vi "UHR-Fleezers Control (host) - 12.6.1.vi"() -> ()   [LabVIEW 2012] (continued)
                    n401 = property on="Saved AOD Raster Scan Parameter Sets" class="Arr (strict)"("Index Values"=w674) -> ()  [unwired: 2 in, 2 out]
                  }
                  frame #1 {
                    n402 = Wait (ms)(milliseconds to wait=u32 200) -> ()  [unwired: 1 out]
                  }
                  frame #2 {
                    n403 = property on="Load parameters" class="Bool (strict)"("Val(Sgnl)"=TRUE ("Value (Signaling)")) -> ()  [unwired: 2 in, 2 out]
                  }
                  frame #3 {
                    n404 = Wait (ms)(milliseconds to wait=u32 200) -> ()  [unwired: 1 out]
                  }
                  frame #4 {
                    n405 = property on="Trap Raster Scan" class="Bool (strict)"("Val(Sgnl)"=TRUE ("Value (Signaling)")) -> ()  [unwired: 2 in, 2 out]
                  }
                  frame #5 {
                    n406 = Wait (ms)(milliseconds to wait=u32 2000) -> ()  [unwired: 1 out]
                  }
                  frame #6 {
                    n407 = while {
                      stop <- w687 stop-if-true
                      n408 = local read "Raster Scanning..."() -> (w689:bool)
                      n409 = local read "Saving..."() -> (w685:bool)
                      n410 = Wait (ms)(milliseconds to wait=u32 100) -> ()  [unwired: 1 out]
                      n411 = Not(x=w685) -> (.not. x?=w684:bool)
                      n412 = Not(x=w689) -> (.not. x?=w686:bool)
                      n413 = And(x=w686, y=w684) -> (x .and. y?=w687:bool)
                    }
                  }
                  frame #7 {
                    n414 = property on="Trap Delta (MHz)" class="DigNum (strict)"("Val(Sgnl)"=w690) -> ()  [unwired: 2 in, 2 out]
                  }
                }
              }
            }
          }
          frame #8 {
            n415 = local read "Save ave N"() -> (w692:dbl)
            n416 = case shown="False" "W/ Offset 2" {
              tunnel: w693 -> [_ w700]
              tunnel: w692 -> [_ w699]
              tunnel: w691 -> [w695 _]
              frame False {
                n417 = case shown="False" w695 {
                  frame False {
                    n418 = Multiply(x="Cal read wait (s)", y=u32 1000 ("milliseconds to wait")) -> (x*y=w697:u32)
                    n419 = Wait (ms)(milliseconds to wait=w697) -> ()  [unwired: 1 out]
                  }
                  frame True {
                  }
                }
              }
              frame True {
                n420 = stacked-sequence {
                  tunnel: w700 -> [_ _ _ _ _ _ _ _ _ w721 _ _]
                  tunnel: w699 -> [_ _ _ _ _ _ _ _ _ w719 _ _]
                  frame #0 {
                    n421 = property on="Save ave N" class="DigNum (strict)"("Val(Sgnl)"=1.0 ("Value (Signaling)")) -> ()  [unwired: 2 in, 2 out]
                  }
                  frame #1 {
                    n422 = Wait (ms)(milliseconds to wait=u32 500) -> ()  [unwired: 1 out]
                  }
                  frame #2 {
                    n423 = property on="Trap Delta (MHz)" class="DigNum (strict)"("Val(Sgnl)"="Offset 2 Start (MHz)") -> ()  [unwired: 2 in, 2 out]
                    n424 = Replace Array Subset(array=u32[] [0] ("Index Values"), new element="Offset 2 Set", index=0) -> (w705:u32[])
                    n425 = property on="Saved AOD Raster Scan Parameter Sets" class="Arr (strict)"("Index Values"=w705) -> ()  [unwired: 2 in, 2 out]
                  }
                  frame #3 {
                    n426 = Wait (ms)(milliseconds to wait=u32 500) -> ()  [unwired: 1 out]
                  }
                  frame #4 {
                    n427 = property on="Load parameters" class="Bool (strict)"("Val(Sgnl)"=TRUE ("Value (Signaling)")) -> ()  [unwired: 2 in, 2 out]
                  }
                  frame #5 {
                    n428 = Wait (ms)(milliseconds to wait=u32 500) -> ()  [unwired: 1 out]
                  }
                  frame #6 {
                    n429 = property on="Trap Raster Scan" class="Bool (strict)"("Val(Sgnl)"=TRUE ("Value (Signaling)")) -> ()  [unwired: 2 in, 2 out]
                  }
                  frame #7 {
                    n430 = Wait (ms)(milliseconds to wait=u32 2000) -> ()  [unwired: 1 out]
                  }
                  frame #8 {
                    n431 = while {
                      stop <- w714 stop-if-true
                      n432 = local read "Raster Scanning..."() -> (w717:bool)
                      n433 = local read "Saving..."() -> (w715:bool)
                      n434 = Wait (ms)(milliseconds to wait=u32 100) -> ()  [unwired: 1 out]
                      n435 = Not(x=w715) -> (.not. x?=w713:bool)
                      n436 = Not(x=w717) -> (.not. x?=w716:bool)
                      n437 = And(x=w716, y=w713) -> (x .and. y?=w714:bool)
                    }
                  }
                  frame #9 {
                    n438 = property on="Trap Delta (MHz)" class="DigNum (strict)"("Val(Sgnl)"=w721) -> ()  [unwired: 2 in, 2 out]
                    n439 = property on="Saved AOD Raster Scan Parameter Sets" class="Arr (strict)"("Index Values"=u32[] [0]) -> ()  [unwired: 2 in, 2 out]
                    n440 = property on="Save ave N" class="DigNum (strict)"("Val(Sgnl)"=w719) -> ()  [unwired: 2 in, 2 out]
                  }
                  frame #10 {
                    n441 = Wait (ms)(milliseconds to wait=u32 500) -> ()  [unwired: 1 out]
                  }
                  frame #11 {
                    n442 = property on="Load parameters" class="Bool (strict)"("Val(Sgnl)"=TRUE ("Value (Signaling)")) -> ()  [unwired: 2 in, 2 out]
                  }
                }
              }
            }
          }
          frame #9 {
            n443 = property on="Read Cal" class="Bool (strict)"("Val(Sgnl)"=TRUE ("Value (Signaling)")) -> ()  [unwired: 2 in, 2 out]
          }
          frame #10 {
            n444 = Wait (ms)(milliseconds to wait=u32 1000) -> ()  [unwired: 1 out]
          }
          frame #11 {
            n445 = property on="Fish for Tether" class="Bool (strict)"("Val(Sgnl)"=TRUE ("Value (Signaling)")) -> ()  [unwired: 2 in, 2 out]
          }
        }
        n446 = local write "Cal/Data Acq. Spot"(FALSE ("Cal/Data Acq. Spot")) -> ()
      }
      event "Dump Beads": Value Change {
        n447 = event-data() -> ()  [unwired: 1 in, 5 out]
        n448 = flat-sequence {
          tunnel: ["Dump spot flow on?"] -> w727
          tunnel: [w738] -> w728
          tunnel: w727 -> [w738]
          tunnel: w731 -> [w743]
          tunnel: w730 -> [w742]
          tunnel: [w740] -> w729
          tunnel: w728 -> [w740]
          tunnel: w729 -> [w753]
          frame #0 {
            w732 = FALSE ("Value (Signaling)")
            n449 = local read "Saving..."() -> (w734:bool)
            n450 = local write "Dump Beads"(FALSE ("Dump Beads")) -> ()
            n451 = property on="Inject Pump 3" class="Bool (strict)"("Val(Sgnl)"=w732) -> ()  [unwired: 2 in, 2 out]
            n452 = property on="Inject Pump 1" class="Bool (strict)"("Val(Sgnl)"=w732) -> ()  [unwired: 2 in, 2 out]
            n453 = local write "Stop Saving"(w734) -> ()
          }
          frame #1 {
            w735 = FALSE ("Fl. Triggered...")
            n454 = case shown="True" "Dump spot flow on?" {
              frame False {
              }
              frame True {
                n455 = property on="Sample Channel\nFlow" class="Bool (strict)"("Val(Sgnl)"=TRUE ("Stage Moving")) -> ()  [unwired: 2 in, 2 out]
              }
            }
            n456 = local write "Fl. Triggered..."(w735) -> ()
            n457 = local write "Tether"(w735) -> ()
            n458 = property on="Green Laser ON" class="Bool (strict)"("Val(Sgnl)"=w735) -> ()  [unwired: 2 in, 2 out]
            n459 = property on="Trap Pos. FB ON" class="Bool (strict)"("Val(Sgnl)"=w735) -> ()  [unwired: 2 in, 2 out]
            n460 = property on="Trap Trig. Fl." class="Bool (strict)"("Val(Sgnl)"=w735) -> ()  [unwired: 2 in, 2 out]
            n461 = property on="Fl. Triggered..." class="Bool (strict)"("Val(Sgnl)"=w735) -> ()  [unwired: 2 in, 2 out]
            n462 = property on="Dip for Protein" class="Bool (strict)"("Val(Sgnl)"=w735) -> ()  [unwired: 2 in, 2 out]
            n463 = property on="Pause dwell" class="Bool (strict)"("Val(Sgnl)"=w735) -> ()  [unwired: 2 in, 2 out]
          }
          frame #2 {
            n464 = property on="Trap Pos. FB Offset Factor" class="DigNum (strict)"("Val(Sgnl)"=i64 0 ("Value (Signaling)")) -> ()  [unwired: 2 in, 2 out]
          }
          frame #3 {
            n465 = local read "Saved Stage Positions"() -> (w744:dbl[][])
            n466 = local write "Stage Moving"(TRUE ("Stage Moving")) -> ()
            n467 = Array Subset(array=w744, index (row)=3 ("index"), length (row)=1 ("length"), index (col)=1 ("index"), length (col)=3 ("length")) -> (w749:dbl[][])
            n468 = Reshape Array(w749, 3 ("dimension size")) -> (w747:dbl[])
            n469 = Array To Cluster(array=w747) -> (cluster=w746:cluster{"[0]":dbl, "[1]":dbl, "[2]":dbl})
            n470 = call "Set Stage Position.vi"("Position"=w746, "error in"=w742, "VISA resource name in"=w743) -> ()  [unwired: 3 out]
          }
          frame #4 {
            w754 = FALSE ("Value (Signaling)")
            n471 = case shown="True" w753 {
              frame False {
              }
              frame True {
                n472 = property on="Sample Channel\nFlow" class="Bool (strict)"("Val(Sgnl)"=FALSE ("Stage Moving")) -> ()  [unwired: 2 in, 2 out]
              }
            }
            n473 = property on="Trap 1 (ON/OFF)" class="Bool (strict)"("Val(Sgnl)"=w754) -> ()  [unwired: 2 in, 2 out]
            n474 = property on="Trap 2 (ON/OFF)" class="Bool (strict)"("Val(Sgnl)"=w754) -> ()  [unwired: 2 in, 2 out]
            n475 = call <vilib>:"Beep.vi"() -> ()  [unwired: 3 in, 9 out]
          }
          frame #5 {
            n476 = property on="Move Cap. 2 (ADig Top)" class="Bool (strict)"("Val(Sgnl)"=TRUE ("Value (Signaling)")) -> ()  [unwired: 2 in, 2 out]
            n477 = property on="Tab Control" class="TabCtl (strict)"("Val(Sgnl)"=T26."Status" ("Value (Signaling)")) -> ()  [unwired: 2 in, 2 out]
          }
        }
      }
      event "Dip for Protein": Value Change {
        n478 = event-data() -> ()  [unwired: 1 in, 5 out]
        n479 = case shown="True" "Dip for Protein" {
          tunnel: w760 -> [_ w762]
          tunnel: w759 -> [_ w761]
          frame False {
          }
          frame True {
            n480 = while {
              tunnel: w762 -> [w773]
              tunnel: w761 -> [w772]
              i -> [w767]
              stop <- w769 stop-if-true
              n481 = Increment(x=w767) -> (x+1=→"Dip #":i32)
              n482 = flat-sequence {
                tunnel: w772 -> [w784]
                tunnel: w773 -> [w785]
                tunnel: [w785] -> w777
                tunnel: [w784] -> w776
                tunnel: [w778] -> w763
                tunnel: [w790] -> w771
                tunnel: [w791] -> w770
                tunnel: w777 -> [w792]
                tunnel: w776 -> [w793]
                tunnel: [w788] -> w764
                tunnel: w763 -> [w788]
                tunnel: [w801] -> w775
                tunnel: w771 -> [w801]
                tunnel: [w800] -> w774
                tunnel: w770 -> [w800]
                tunnel: [w797] -> w768
                tunnel: [w796] -> w765
                tunnel: w764 -> [w796]
                tunnel: w774 -> [w821]
                tunnel: w775 -> [w822]
                tunnel: w768 -> [w823]
                tunnel: w765 -> [w820]
                tunnel: [w879] -> w769
                frame #0 {
                  n483 = local read "Trap Pos. FB ON"() -> (w778:bool)
                  n484 = Compound Arithmetic op=AND("Flow ON\nduring dip?", "FB OFF when \nflow ON", w778) -> (w779:bool)
                  n485 = case shown="True" "Move trap \nbefore dip move?" {
                    frame False {
                    }
                    frame True {
                      n486 = property on="Trap Delta (MHz)" class="DigNum (strict)"("Val(Sgnl)"="Dipping Delta (MHz)") -> ()  [unwired: 2 in, 2 out]
                    }
                  }
                  n487 = property on="Green Laser ON" class="Bool (strict)"("Val(Sgnl)"="Green ON\nbefore dip?") -> ()  [unwired: 2 in, 2 out]
                  n488 = property on="Sample Channel\nFlow" class="Bool (strict)"("Val(Sgnl)"="Flow ON\nduring dip?") -> ()  [unwired: 2 in, 2 out]
                  n489 = case shown="True" w779 {
                    frame False {
                    }
                    frame True {
                      n490 = property on="Trap Pos. FB ON" class="Bool (strict)"("Val(Sgnl)"=FALSE ("Value (Signaling)")) -> ()  [unwired: 2 in, 2 out]
                    }
                  }
                }
                frame #1 {
                  n491 = local read "Saved Stage Positions"() -> (w795:dbl[][])
                  n492 = local write "Cancel dwell"(FALSE ("Cancel dwell")) -> ()
                  n493 = call "move to saved stage position.vi"("error in"=w793, "Stage VISA resource name in"=w792, "Position"="Dip Stage \nPosition", "Saved Stage Positions"=w795) -> ("VISA resource name out"=w790:refnum<visa-resource-name>, "error out"=w791:errorcluster)
                }
                frame #2 {
                  n494 = node-c288() -> (w799:T23)  [unwired: 4 in]
                  n495 = timed-loop {
                    timing: w799 -> [_]
                    timing-out: [_] -> w798
                    tunnel: [w805] -> w797
                    i -> [w802]
                    stop <- w806 stop-if-true
                    n496 = node-c288() -> ()  [unwired: 1 in, 1 out]
                    n497 = Greater Or Equal?(x=w802, y="Dip Duration (s)") -> (x >= y?=w814:bool)
                    n498 = local read "Dip for Protein"() -> (w807:bool)
                    n499 = local read "Dump Beads"() -> (w804:bool)
                    n500 = local read "Cancel dwell"() -> (w813:bool)
                    n501 = local read "Pause dwell"() -> (w810:bool)
                    n502 = Not(x=w807) -> (.not. x?=w812:bool)
                    n503 = Compound Arithmetic op=OR(w813, w814, w812) -> (w811:bool)
                    n504 = Select(t=FALSE, s=w810, f=w811) -> (s? t:f=w808:bool)
                    n505 = Not(x=w804) -> (.not. x?=w803:bool)
                    n506 = node-c288() -> ()  [unwired: 1 in, 1 out]
                    n507 = And(x=w807, y=w803) -> (x .and. y?=w805:bool)
                    n508 = Or(x=w808, y=w804) -> (x .or. y?=w806:bool)
                    "Dip Time (s)" <- w802
                  }
                  n509 = node-c288(w798) -> ()  [unwired: 1 out]
                }
                frame #3 {
                  n510 = case shown="True" w823 {
                    tunnel: w822 -> [_ w828]
                    tunnel: w821 -> [_ w827]
                    tunnel: w820 -> [_ w824]
                    frame False {
                    }
                    frame True {
                      n511 = flat-sequence {
                        tunnel: w827 -> [w832]
                        tunnel: w828 -> [w833]
                        tunnel: [w833] -> w826
                        tunnel: [w832] -> w825
                        tunnel: w824 -> [w829]
                        tunnel: w826 -> [w843]
                        tunnel: w825 -> [w842]
                        tunnel: w824 -> [w851]
                        frame #0 {
                          n512 = local read "Sample Channel\nFlow"() -> (w831:bool)
                          n513 = case shown="True" w831 {
                            tunnel: "Flow ON \nduring return\nfrom dip?" -> [w834 w837]
                            tunnel: w829 -> [_ w836]
                            frame False {
                              n514 = case shown="True" w834 {
                                frame False {
                                }
                                frame True {
                                n515 = property on="Sample Channel\nFlow" class="Bool (strict)"("Val(Sgnl)"=TRUE ("Value (Signaling)")) -> ()  [unwired: 2 in, 2 out]
                                }
                              }
                            }
                            frame True {
                              n516 = case shown="False" w837 {
                                tunnel: w836 -> [w838 _]
                                frame False {
                                n517 = property on="Trap Pos. FB ON" class="Bool (strict)"("Val(Sgnl)"=w838) -> ()  [unwired: 2 in, 2 out]
                                n518 = property on="Sample Channel\nFlow" class="Bool (strict)"("Val(Sgnl)"=FALSE ("Value (Signaling)")) -> ()  [unwired: 2 in, 2 out]
                                }
                                frame True {
                                }
                              }
                            }
                          }
                        }
                        frame #1 {
                          # "For turning on green laser before stage reaches lower spot"
                          n519 = case shown="True" "Green ON\nafter start\nreturn?" {
                            frame False {
                            }
                            frame True {
                              n520 = flat-sequence {
                                frame #0 {
                                n521 = Multiply(x="Green delay after \nstart return (s)", y=1000.0) -> (x*y=w848:dbl)
                                n522 = Wait (ms)(milliseconds to wait=w848) -> ()  [unwired: 1 out]
                                }
                                frame #1 {
                                n523 = property on="Green Laser ON" class="Bool (strict)"("Val(Sgnl)"=TRUE ("Value (Signaling)")) -> ()  [unwired: 2 in, 2 out]
                                }
                              }
                            }
                          }
                          n524 = local read "Saved Stage Positions"() -> (w846:dbl[][])
                          n525 = local write "Cancel dwell"(FALSE ("Cancel dwell")) -> ()
                          n526 = call "move to saved stage position.vi"("error in"=w842, "Stage VISA resource name in"=w843, "Position"="Return Stage \nPosition", "Saved Stage Positions"=w846) -> ("error out"=w844:errorcluster)  [unwired: 1 out]
                          n527 = local write "Stage Control Serial Error"(w844) -> ()
                        }
                        frame #2 {
                          n528 = property on="Trap Pos. FB ON" class="Bool (strict)"("Val(Sgnl)"=w851) -> ()  [unwired: 2 in, 2 out]
                          n529 = case shown="True" "Green ON \nafter return?" {
                            frame False {
                            }
                            frame True {
                              n530 = property on="Green Laser ON" class="Bool (strict)"("Val(Sgnl)"=TRUE ("Value (Signaling)")) -> ()  [unwired: 2 in, 2 out]
                            }
                          }
                          n531 = case shown="True" "Move trap after return?" {
                            frame False {
                            }
                            frame True {
                              n532 = property on="Trap Delta (MHz)" class="DigNum (strict)"("Val(Sgnl)"="Dip Trap Delta 2 (MHz)") -> ()  [unwired: 2 in, 2 out]
                            }
                          }
                          n533 = case shown="True" "Save data after return?" {
                            frame False {
                            }
                            frame True {
                              n534 = property on="Start Saving" class="Bool (strict)"("Val(Sgnl)"=TRUE ("Value (Signaling)")) -> ()  [unwired: 2 in, 2 out]
                            }
                          }
                          n535 = property on="Sample Channel\nFlow" class="Bool (strict)"("Val(Sgnl)"="Flow ON\nduring daq?") -> ()  [unwired: 2 in, 2 out]
                        }
                        frame #3 {
                          n536 = node-c288() -> (w860:T23)  [unwired: 4 in]
                          n537 = timed-loop {
                            timing: w860 -> [_]
                            timing-out: [_] -> w859
                            i -> [w861]
                            stop <- w863 stop-if-true
                            n538 = node-c288() -> ()  [unwired: 1 in, 1 out]
                            n539 = local read "Dump Beads"() -> (w862:bool)
                            n540 = Greater Or Equal?(x=w861, y="Dwell Duration (s)") -> (x >= y?=w868:bool)
                            n541 = local read "Dip for Protein"() -> (w865:bool)
                            n542 = Not(x=w865) -> (.not. x?=w864:bool)
                            n543 = Compound Arithmetic op=OR(w868, "Cancel dwell", w864) -> (w867:bool)
                            n544 = node-c288() -> ()  [unwired: 1 in, 1 out]
                            n545 = Select(t=FALSE, s="Pause dwell", f=w867) -> (s? t:f=w870:bool)
                            n546 = Or(x=w870, y=w862) -> (x .or. y?=w863:bool)
                            "Dwell Time (s)" <- w861
                          }
                          n547 = node-c288(w859) -> ()  [unwired: 1 out]
                        }
                      }
                    }
                  }
                }
                frame #4 {
                  n548 = local read "Dip for Protein"() -> (w880:bool)
                  n549 = local read "Dump Beads"() -> (w877:bool)
                  n550 = local write "Cancel dwell"(FALSE ("Cancel dwell")) -> ()
                  n551 = Not(x=w880) -> (.not. x?=w881:bool)
                  n552 = Not(x="Cont. Repeat Dipping?") -> (.not. x?=w883:bool)
                  n553 = Compound Arithmetic op=OR(w881, w883, w877) -> (w879:bool)
                }
              }
            }
          }
        }
      }
      event "Profile": Value Change {
        n554 = event-data() -> ()  [unwired: 1 in, 5 out]
        n555 = flat-sequence {
          tunnel: w892 -> [w895]
          tunnel: w891 -> [w903]
          tunnel: [w897] -> w890
          tunnel: [w896] -> w889
          tunnel: [w894] -> w887
          tunnel: [w893] -> w884
          tunnel: w890 -> [w910]
          tunnel: w889 -> [w909]
          tunnel: [w907] -> w888
          tunnel: w887 -> [w908]
          tunnel: [w906] -> w886
          tunnel: [w905] -> w885
          tunnel: w884 -> [w905]
          tunnel: w888 -> [w914]
          tunnel: w886 -> [w913]
          tunnel: w885 -> [w912]
          frame #0 {
            n556 = call "Read Stage Position.vi"("error in"=w903, "VISA resource name in"=w895) -> ("Current Position"=w893:cluster{dbl, dbl, dbl}, "error out"=w896:errorcluster, "VISA resource name out"=w894:refnum<visa-resource-name>)  [unwired: 1 out]
            "Current Position" <- w893
            n557 = local write "Stage Control Serial Error"(w896) -> ()
            n558 = Unbundle(w893) -> (w900:dbl, w902:dbl, w898:dbl)
            n559 = Add(x=w902, y="Y change (mm)") -> (x+y=w899:dbl)
            n560 = Bundle(w900, w899, w898) -> (w897:cluster{dbl, dbl, dbl})  [unwired: 1 in]
          }
          frame #1 {
            # "move to new position and start saving"
            n561 = local write "Stage Moving"(TRUE ("Stage Moving")) -> ()
            n562 = local write "Start Saving"(TRUE ("Start Saving")) -> ()
            n563 = call "Set Stage Position.vi"("Position"=w910, "error in"=w909, "VISA resource name in"=w908) -> ("error out"=w906:errorcluster, "VISA resource name out"=w907:refnum<visa-resource-name>)  [unwired: 1 out]
          }
          frame #2 {
            # "go back to start"
            n564 = call "Set Stage Position.vi"("Position"=w912, "error in"=w913, "VISA resource name in"=w914) -> ()  [unwired: 3 out]
          }
          frame #3 {
            # "stop saving"
            n565 = local write "Stop Saving"(TRUE ("Stop Saving")) -> ()
            n566 = local write "Stage Moving"(FALSE ("Stage Moving")) -> ()
          }
        }
      }
      event "Move to Position 1", "Move to Position 2", "Move to Position 3", "Move to Position 4", "Move to Position 5", "Lower Ch. Cap.": Value Change {
        n567 = event-data() -> ()  [unwired: 1 in, 5 out]
        n568 = Or(x="Move to Position 5", y="Lower Ch. Cap.") -> (x .or. y?=w920:bool)
        n569 = Build Array("Move to Position 1", "Move to Position 2", "Move to Position 3", "Move to Position 4", w920) -> (w923:bool[])
        n570 = Boolean Array To Number(Boolean array=w923) -> (number=w922:u32)
        n571 = Logarithm Base 2(1:w922) -> (0:w921:dbl)
        n572 = flat-sequence {
          tunnel: w921 -> [w932]
          tunnel: w918 -> [w930]
          tunnel: w917 -> [w929]
          frame #0 {
            n573 = local read "Saved Stage Positions"() -> (w940:dbl[][])
            n574 = Array Subset(array=w940, index (row)=w932, length (row)=1 ("length"), index (col)=1 ("index"), length (col)=3 ("length")) -> (w937:dbl[][])
            n575 = Reshape Array(w937, 3 ("dimension size")) -> (w935:dbl[])
            n576 = Array To Cluster(array=w935) -> (cluster=w934:cluster{"[0]":dbl, "[1]":dbl, "[2]":dbl})
            n577 = call "Set Stage Position.vi"("Position"=w934, "error in"=w929, "VISA resource name in"=w930) -> ("error out"=w933:errorcluster)  [unwired: 2 out]
            n578 = local write "Stage Moving"(TRUE ("Stage Moving")) -> ()
            n579 = local write "Stage Control Serial Error"(w933) -> ()
          }
          frame #1 {
            n580 = local write "Stage Moving"(FALSE ("Stage Moving")) -> ()
            n581 = call <vilib>:"Beep.vi"() -> ()  [unwired: 3 in, 9 out]
          }
        }
      }
      event "Got ADig bead": Value Change {
        n582 = event-data() -> ()  [unwired: 1 in, 5 out]
        n583 = flat-sequence {
          frame #0 {
            n584 = local read "Cap 1 Samp Flow ON"() -> (w944:bool)
            n585 = case shown="True" w944 {
              frame False {
              }
              frame True {
                n586 = property on="Sample Channel\nFlow" class="Bool (strict)"("Val(Sgnl)"=TRUE ("Value (Signaling)")) -> ()  [unwired: 2 in, 2 out]
              }
            }
          }
          frame #1 {
            n587 = property on="Inject Pump 3" class="Bool (strict)"("Val(Sgnl)"=FALSE ("Value (Signaling)")) -> ()  [unwired: 2 in, 2 out]
          }
          frame #2 {
            n588 = property on="Move Cap. 1 (DNA Bottom)" class="Bool (strict)"("Val(Sgnl)"=TRUE ("Value (Signaling)")) -> ()  [unwired: 2 in, 2 out]
          }
        }
      }
      event "Force FB Data\nScript": Value Change {
        n589 = event-data() -> ()  [unwired: 1 in, 5 out]
        n590 = flat-sequence {
          tunnel: w953 -> [w957]
          tunnel: w954 -> [w958]
          tunnel: [w958] -> w949
          tunnel: [w957] -> w948
          tunnel: w949 -> [w961]
          tunnel: w948 -> [w960]
          tunnel: ["Trap Trig Fl."] -> w950
          tunnel: [w986] -> w951
          tunnel: w950 -> [w986]
          tunnel: [w990] -> w952
          tunnel: w951 -> [w990]
          tunnel: w952 -> [w992]
          frame #0 {
            n591 = property on="Trap Delta (MHz)" class="DigNum (strict)"("Val(Sgnl)"="Trap Delta Before Moving") -> ()  [unwired: 2 in, 2 out]
          }
          frame #1 {
            n592 = local read "Saved Stage Positions"() -> (w963:dbl[][])
            n593 = local write "FB Trap Pos Offset"(0.0 ("FB Trap Pos Offset")) -> ()
            n594 = property on="Trap Pos. FB Offset Factor" class="DigNum (strict)"("Val(Sgnl)"=i64 0 ("Value (Signaling)")) -> ()  [unwired: 2 in, 2 out]
            n595 = local write "Stage Moving"(TRUE ("Stage Moving")) -> ()
            n596 = call "move to saved stage position.vi"("error in"=w960, "Stage VISA resource name in"=w961, "Position"="Stage Position To Establish FB", "Saved Stage Positions"=w963) -> ("error out"=w959:errorcluster)  [unwired: 1 out]
            n597 = local write "Stage Control Serial Error"(w959) -> ()
          }
          frame #2 {
            n598 = call <vilib>:"Beep.vi"() -> ()  [unwired: 3 in, 9 out]
            n599 = Multiply(x="Wait (s)", y=u32 1000 ("milliseconds to wait")) -> (x*y=w970:u32)
            n600 = property on="Trap Delta (MHz)" class="DigNum (strict)"("Val(Sgnl)"="Starting \nTrap Delta (MHz)") -> ()  [unwired: 2 in, 2 out]
            n601 = local write "Stage Moving"(FALSE ("Stage Moving")) -> ()
            n602 = Wait (ms)(milliseconds to wait=w970) -> ()  [unwired: 1 out]
            n603 = property on="Tab Control 2" class="TabCtl (strict)"("Val(Sgnl)"=T6."Feedback on Trap Position" ("Value (Signaling)")) -> ()  [unwired: 2 in, 2 out]
            n604 = property on="Tab Control" class="TabCtl (strict)"("Val(Sgnl)"=T27."Trap Control (RF)" ("Value (Signaling)")) -> ()  [unwired: 2 in, 2 out]
          }
          frame #3 {
            n605 = property on="Set Reading to\nSetpoint" class="Bool (strict)"("Val(Sgnl)"=TRUE ("Value (Signaling)")) -> ()  [unwired: 2 in, 2 out]
            n606 = Wait (ms)(milliseconds to wait=u32 500) -> ()  [unwired: 1 out]
          }
          frame #4 {
            n607 = property on="Trap Pos. FB ON" class="Bool (strict)"("Val(Sgnl)"=TRUE ("Value (Signaling)")) -> ()  [unwired: 2 in, 2 out]
            n608 = Wait (ms)(milliseconds to wait=u32 250) -> ()  [unwired: 1 out]
          }
          frame #5 {
            n609 = case shown="False" "Trap Trig Fl." {
              frame False {
                n610 = case shown="True" "Green ON after FB ON?" {
                  selector: "Green ON after FB ON?" -> [_ w985]
                  frame False {
                  }
                  frame True {
                    n611 = property on="Green Laser ON" class="Bool (strict)"("Val(Sgnl)"=w985) -> ()  [unwired: 2 in, 2 out]
                  }
                }
              }
              frame True {
              }
            }
            n612 = case shown="True" "Remove Action Offset" {
              tunnel: TRUE ("Value (Signaling)") -> [w982 w983]
              frame False {
                n613 = property on="Remove Unwinding Offset" class="Bool (strict)"("Val(Sgnl)"=w982) -> ()  [unwired: 2 in, 2 out]
              }
              frame True {
                n614 = property on="Remove Action Offset" class="Bool (strict)"("Val(Sgnl)"=w983) -> ()  [unwired: 2 in, 2 out]
              }
            }
            n615 = Wait (ms)(milliseconds to wait=u32 250) -> ()  [unwired: 1 out]
          }
          frame #6 {
            n616 = property on="Start Saving" class="Bool (strict)"("Val(Sgnl)"=TRUE ("Value (Signaling)")) -> ()  [unwired: 2 in, 2 out]
            n617 = Wait (ms)(milliseconds to wait=u32 5000) -> ()  [unwired: 1 out]
          }
          frame #7 {
            w989 = TRUE ("Value (Signaling)")
            n618 = property on="Rem fb disp offset" class="Bool (strict)"("Val(Sgnl)"=w989) -> ()  [unwired: 2 in, 2 out]
            n619 = property on="Remove Offset" class="Bool (strict)"("Val(Sgnl)"=w989) -> ()  [unwired: 2 in, 2 out]
            n620 = Wait (ms)(milliseconds to wait=u32 100) -> ()  [unwired: 1 out]
          }
          frame #8 {
            n621 = case shown="True" w992 {
              frame False {
              }
              frame True {
                n622 = local write "Trap Trig. Fl."(TRUE ("Value (Signaling)")) -> ()
              }
            }
          }
          frame #9 {
            n623 = case shown="True" "Start dipping after?" {
              frame False {
              }
              frame True {
                n624 = flat-sequence {
                  frame #0 {
                    n625 = Multiply(x="Delay before dipping (s)", y=1000.0) -> (x*y=w996:dbl)
                    n626 = Wait (ms)(milliseconds to wait=w996) -> ()  [unwired: 1 out]
                  }
                  frame #1 {
                    n627 = property on="Dip for Protein" class="Bool (strict)"("Val(Sgnl)"=TRUE ("Value (Signaling)")) -> ()  [unwired: 2 in, 2 out]
                    n628 = local write "Scripts"(T1."Dipping" ("Scripts")) -> ()
                  }
                }
              }
            }
          }
        }
      }
      event "Fixed Traps Data\nScript": Value Change {
        n629 = event-data() -> ()  [unwired: 1 in, 5 out]
        n630 = flat-sequence {
          frame #0 {
            n631 = case shown="True" "Green ON" {
              frame False {
              }
              frame True {
                n632 = property on="Green Laser ON" class="Bool (strict)"("Val(Sgnl)"=TRUE) -> ()  [unwired: 2 in, 2 out]
              }
            }
            n633 = local write "Offset (nm)"(0.0 ("Offset (nm)")) -> ()
            n634 = property on="Sample Channel\nFlow" class="Bool (strict)"("Val(Sgnl)"=FALSE ("Value (Signaling)")) -> ()  [unwired: 2 in, 2 out]
            n635 = property on="Trap Delta (MHz)" class="DigNum (strict)"("Val(Sgnl)"="Fixed Traps Trap Delta (MHz)") -> ()  [unwired: 2 in, 2 out]
          }
          frame #1 {
            n636 = Wait (ms)(milliseconds to wait=u32 1000) -> ()  [unwired: 1 out]
          }
          frame #2 {
            n637 = local write "Start Saving"(TRUE ("Start Saving")) -> ()
          }
          frame #3 {
            n638 = local read "Bead Sep. Int. Time (s)"() -> (w1007:dbl)
            n639 = Multiply(x=w1007, y=1000.0) -> (x*y=w1009:dbl)
            n640 = Wait (ms)(milliseconds to wait=w1009) -> ()  [unwired: 1 out]
          }
          frame #4 {
            n641 = property on="Remove Offset" class="Bool (strict)"("Val(Sgnl)"=TRUE ("Value (Signaling)")) -> ()  [unwired: 2 in, 2 out]
          }
          frame #5 {
            n642 = property on="Dip for Protein" class="Bool (strict)"("Val(Sgnl)"="Start dipping after?") -> ()  [unwired: 2 in, 2 out]
          }
        }
      }
      event "Got DNA bead": Value Change {
        n643 = event-data() -> ()  [unwired: 1 in, 5 out]
        n644 = flat-sequence {
          frame #0 {
            n645 = local read "Daq spot flow on"() -> (w1014:bool)
            n646 = case shown="True" w1014 {
              frame False {
              }
              frame True {
                n647 = property on="Sample Channel\nFlow" class="Bool (strict)"("Val(Sgnl)"=TRUE ("Value (Signaling)")) -> ()  [unwired: 2 in, 2 out]
              }
            }
            n648 = property on="Got DNA bead" class="Bool"("Key Focus"=FALSE) -> ()  [unwired: 2 in, 2 out]
          }
          frame #1 {
            n649 = property on="Inject Pump 1" class="Bool (strict)"("Val(Sgnl)"=FALSE ("Value (Signaling)")) -> ()  [unwired: 2 in, 2 out]
          }
          frame #2 {
            n650 = property on="Cal/Data Acq. Spot" class="Bool (strict)"("Val(Sgnl)"=TRUE ("Value (Signaling)")) -> ()  [unwired: 2 in, 2 out]
          }
        }
      }
      event "Take Stepping Data": Value Change {
        n651 = event-data() -> ()  [unwired: 1 in, 5 out]
        n652 = local read "Save ave N"() -> (w1026:dbl)
        n653 = flat-sequence {
          tunnel: w1026 -> [w1028]
          tunnel: [w1028] -> w1021
          tunnel: [w1030] -> w1022
          tunnel: w1021 -> [w1030]
          tunnel: [w1032] -> w1023
          tunnel: w1022 -> [w1032]
          tunnel: [w1035] -> w1024
          tunnel: w1023 -> [w1035]
          tunnel: [w1037] -> w1025
          tunnel: w1024 -> [w1037]
          tunnel: [w1039] -> w1019
          tunnel: w1025 -> [w1039]
          tunnel: w1019 -> [w1042]
          tunnel: [w1042] -> w1018
          tunnel: w1018 -> [w1043]
          tunnel: [w1043] -> w1020
          tunnel: w1020 -> [w1049]
          frame #0 {
            n654 = property on="Save ave N" class="DigNum (strict)"("Val(Sgnl)"="Save ave factor") -> ()  [unwired: 2 in, 2 out]
          }
          frame #1 {
            n655 = Wait (ms)(milliseconds to wait=u32 100) -> ()  [unwired: 1 out]
          }
          frame #2 {
            n656 = local read "Offset 2 Start (MHz)"() -> (w1034:dbl)
            n657 = property on="Saved AOD Raster Scan Parameter Sets" class="Arr (strict)"("Index Values"=u32[] [2]) -> ()  [unwired: 2 in, 2 out]
            n658 = property on="Trap Delta (MHz)" class="DigNum (strict)"("Val(Sgnl)"=w1034) -> ()  [unwired: 2 in, 2 out]
          }
          frame #3 {
            n659 = property on="Load parameters" class="Bool (strict)"("Val(Sgnl)"=TRUE ("Value (Signaling)")) -> ()  [unwired: 2 in, 2 out]
          }
          frame #4 {
            n660 = Wait (ms)(milliseconds to wait=u32 100) -> ()  [unwired: 1 out]
          }
          frame #5 {
            n661 = property on="Trap Raster Scan" class="Bool (strict)"("Val(Sgnl)"=TRUE ("Value (Signaling)")) -> ()  [unwired: 2 in, 2 out]
          }
          frame #6 {
            n662 = Wait (ms)(milliseconds to wait=u32 1000) -> ()  [unwired: 1 out]
          }
          frame #7 {
            n663 = while {
              stop <- w1046 stop-if-true
              n664 = local read "Raster Scanning..."() -> (w1048:bool)
              n665 = local read "Saving..."() -> (w1047:bool)
              n666 = Not(x=w1047) -> (.not. x?=w1044:bool)
              n667 = Not(x=w1048) -> (.not. x?=w1045:bool)
              n668 = And(x=w1045, y=w1044) -> (x .and. y?=w1046:bool)
            }
          }
          frame #8 {
            n669 = property on="Save ave N" class="DigNum (strict)"("Val(Sgnl)"=w1049) -> ()  [unwired: 2 in, 2 out]
          }
        }
      }
      event "Step Size (nm)": Value Change {
        n670 = event-data() -> ()  [unwired: 1 in, 5 out]
        n671 = flat-sequence {
          frame #0 {
            n672 = property on="Saved AOD Raster Scan Parameter Sets" class="Arr (strict)"("Index Values"=u32[] [1]) -> ()  [unwired: 2 in, 2 out]
          }
          frame #1 {
            n673 = Multiply(x="N Steps", y="Step Size (nm)") -> (x*y=w1051:dbl)
            n674 = property on="Scan Speed AOD (nm/s) 2" class="DigNum (strict)"("Value"="Step Size (nm)") -> ()  [unwired: 2 in, 2 out]
            n675 = property on="Step Size AOD (nm) 2" class="DigNum (strict)"("Value"="Step Size (nm)") -> ()  [unwired: 2 in, 2 out]
            n676 = property on="Scan Range AOD (nm) 2" class="DigNum (strict)"("Value"=w1051) -> ()  [unwired: 2 in, 2 out]
          }
        }
      }
      event "Take Detection Laser\nImage": Value Change {
        n677 = event-data() -> ()  [unwired: 1 in, 5 out]
        n678 = flat-sequence {
          tunnel: [w1079] -> w1069
          tunnel: [w1078] -> w1062
          tunnel: [w1077] -> w1054
          tunnel: [w1082] -> w1070
          tunnel: w1069 -> [w1082]
          tunnel: [w1081] -> w1063
          tunnel: w1062 -> [w1081]
          tunnel: [w1080] -> w1055
          tunnel: w1054 -> [w1080]
          tunnel: [w1086] -> w1071
          tunnel: w1070 -> [w1086]
          tunnel: [w1085] -> w1064
          tunnel: w1063 -> [w1085]
          tunnel: [w1084] -> w1056
          tunnel: w1055 -> [w1084]
          tunnel: [w1092] -> w1072
          tunnel: w1071 -> [w1092]
          tunnel: [w1091] -> w1065
          tunnel: w1064 -> [w1091]
          tunnel: [w1090] -> w1057
          tunnel: w1056 -> [w1090]
          tunnel: [w1096] -> w1073
          tunnel: w1072 -> [w1096]
          tunnel: [w1095] -> w1066
          tunnel: w1065 -> [w1095]
          tunnel: [w1094] -> w1058
          tunnel: w1057 -> [w1094]
          tunnel: [w1100] -> w1074
          tunnel: w1073 -> [w1100]
          tunnel: [w1099] -> w1067
          tunnel: w1066 -> [w1099]
          tunnel: [w1098] -> w1059
          tunnel: w1058 -> [w1098]
          tunnel: [w1104] -> w1075
          tunnel: w1074 -> [w1104]
          tunnel: [w1103] -> w1068
          tunnel: w1067 -> [w1103]
          tunnel: [w1102] -> w1060
          tunnel: w1059 -> [w1102]
          tunnel: w1075 -> [w1110]
          tunnel: w1068 -> [w1109]
          tunnel: [w1107] -> w1061
          tunnel: w1060 -> [w1107]
          tunnel: w1061 -> [w1111]
          frame #0 {
            n679 = local read "Laser interlacing mode"() -> (w1078:enum32{"Laser ON", "Laser OFF", "Interlace"})
            n680 = local read "Green FB On/Off"() -> (w1077:bool)
            n681 = local read "Green Laser ON"() -> (w1079:bool)
          }
          frame #1 {
            n682 = property on="Green FB On/Off" class="Bool (strict)"("Val(Sgnl)"=FALSE ("Value (Signaling)")) -> ()  [unwired: 2 in, 2 out]
          }
          frame #2 {
            n683 = property on="Green Laser ON" class="Bool (strict)"("Val(Sgnl)"=TRUE ("Value (Signaling)")) -> ()  [unwired: 2 in, 2 out]
            n684 = property on="Flip Green Filter" class="Bool (strict)"("Val(Sgnl)"=TRUE ("Value (Signaling)")) -> ()  [unwired: 2 in, 2 out]
            n685 = property on="Laser interlacing mode" class="RadioBtnsControl (strict)"("Val(Sgnl)"=enum32{"Laser ON", "Laser OFF", "Interlace"}."Laser ON" ("Value (Signaling)")) -> ()  [unwired: 2 in, 2 out]
          }
          frame #3 {
            n686 = Wait (ms)(milliseconds to wait=u32 500) -> ()  [unwired: 1 out]
          }
          frame #4 {
            n687 = property on="Confocal Image" class="Bool (strict)"("Val(Sgnl)"=TRUE ("Value (Signaling)")) -> ()  [unwired: 2 in, 2 out]
          }
          frame #5 {
            n688 = Wait (ms)(milliseconds to wait=u32 2000) -> ()  [unwired: 1 out]
          }
          frame #6 {
            n689 = while {
              stop <- w1105 stop-if-true
              n690 = local read "Saving..."() -> (w1106:bool)
              n691 = Not(x=w1106) -> (.not. x?=w1105:bool)
            }
          }
          frame #7 {
            n692 = property on="Flip Green Filter" class="Bool (strict)"("Val(Sgnl)"=TRUE ("Value (Signaling)")) -> ()  [unwired: 2 in, 2 out]
            n693 = property on="Green Laser ON" class="Bool (strict)"("Val(Sgnl)"=w1110) -> ()  [unwired: 2 in, 2 out]
            n694 = property on="Laser interlacing mode" class="RadioBtnsControl (strict)"("Val(Sgnl)"=w1109) -> ()  [unwired: 2 in, 2 out]
          }
          frame #8 {
            n695 = property on="Green FB On/Off" class="Bool (strict)"("Val(Sgnl)"=w1111) -> ()  [unwired: 2 in, 2 out]
          }
        }
      }
      event "Stop All": Value Change {
        # "Stopping blue laser before shutting off program"
        n696 = event-data() -> ()  [unwired: 1 in, 5 out]
        n697 = local read "Delay (ms)"() -> (w1114:i32)
        n698 = call "serial write macro.vi"("String"="l0", "Delay (ms)"=w1114, "VISA resource name"=w1117) -> ("read buffer"=w1112:string, "error out"=w1113:errorcluster, "VISA resource name out"=w1116:refnum<visa-resource-name>)
        n699 = local write "read blue buffer"(w1112) -> ()
        n700 = local write "Blue Error Out"(w1113) -> ()
        n701 = VISA Close(VISA resource name=w1116) -> ()  [unwired: 1 in, 1 out]
        n702 = local read "Stop All"() -> (w1118:bool)
      }
    }
    n703 = node-c288() -> ()  [unwired: 1 in, 1 out]
  }
  n704 = node-c288() -> (w11:T23)  [unwired: 4 out]
  n705 = timed-loop "Oscillate Trap/AOM (fishing, conjugate plane alignment)" {
    tunnel: w17 -> [w1120]
    tunnel: [w1119] -> w130
    timing: w125 -> [_]
    timing-out: [_] -> w124
    stop <- w1119 stop-if-true
    n706 = node-c288() -> ()  [unwired: 2 out]
    n707 = event shown="[0] \"Oscillate Set 1\", \"Fish for Tether\": Value Change" {
      selector: _ -> [_ _ _]
      dyn-events: _ -> [_ _ _]
      timeout: _ -> [_ _ _]
      tunnel: w1120 -> [w1127 _ _]
      tunnel: [FALSE ("Stop All") _ w1725] -> w1119
      event "Oscillate Set 1", "Fish for Tether": Value Change {
        n708 = event-data() -> ()  [unwired: 6 out]
        n709 = local read "Oscillate Set 1"() -> (w1126:bool)
        n710 = Or(x=w1126, y="Fish for Tether") -> (x .or. y?=w1124:bool)
        n711 = case shown="True" w1124 {
          tunnel: w1127 -> [_ w1130]
          tunnel: "Fish for Tether" -> [_ w1129]
          frame False {
          }
          frame True {
            n712 = case shown="True" w1129 {
              selector: w1129 -> [w1133 w1139]
              tunnel: [w1133 w1139] -> w1128
              frame False {
              }
              frame True {
                n713 = local write "Scan axis 2"(TRUE) -> ()
                n714 = local write "Tether"(FALSE ("Tether")) -> ()
                n715 = local read "Flow ON during cal?"() -> (w1134:bool)
                n716 = property on="Trap Delta (MHz)" class="DigNum (strict)"("Val(Sgnl)"="Furthest Delta (MHz)") -> ()  [unwired: 2 in, 2 out]
                n717 = Or(x="Flow ON during \nfishing?", y=w1134) -> (x .or. y?=w1135:bool)
                n718 = Wait (ms)(milliseconds to wait=u32 500) -> ()  [unwired: 1 out]
                n719 = property on="Sample Channel\nFlow" class="Bool (strict)"("Val(Sgnl)"=w1135) -> ()  [unwired: 2 in, 2 out]
              }
            }
            n720 = node-c288() -> (w1132:T23)  [unwired: 1 in, 3 out]
            n721 = timed-loop "Oscillate AOD" {
              timing: w1132 -> [_]
              timing-out: [_] -> w1131
              tunnel: w1130 -> [w1149]
              tunnel: w1128 -> [w1142]
              i -> [w1151]
              stop <- w1148 stop-if-true
              n722 = node-c288() -> (w1150:i64)  [unwired: 1 out]
              n723 = flat-sequence {
                tunnel: w1151 -> [w1178]
                tunnel: w1150 -> [w1177]
                tunnel: w1149 -> [w1159]
                tunnel: w1142 -> [w1161]
                tunnel: [w1161] -> w1147
                tunnel: [w1160] -> w1146
                tunnel: [w1158] -> w1145
                tunnel: [w1155] -> w1143
                tunnel: w1147 -> [w1223]
                tunnel: w1146 -> [w1221]
                tunnel: w1145 -> [w1220]
                tunnel: [w1219] -> w1144
                tunnel: w1143 -> [w1218]
                tunnel: [w1295] -> w1148
                tunnel: w1144 -> [w1294]
                frame #0 {
                  # "w (rad/s)"
                  # "t (s)"
                  n724 = Divide(x=w1177, y=i64 1000) -> (x/y=w1152:dbl)
                  n725 = local read "BD 1 Frequency 2 (MHz)"() -> (w1154:dbl)
                  n726 = Multiply(x="Osc. freq. (Hz)", y=6.283185307179586) -> (x*y=w1175:dbl)
                  n727 = Multiply(x=w1152, y=w1178) -> (x*y=w1174:dbl)
                  n728 = Multiply(x=w1175, y=w1174) -> (x*y=w1157:dbl)
                  n729 = local read "BD 1 Frequency 1 (MHz)"() -> (w1163:dbl)
                  n730 = case shown="True" w1161 {
                    tunnel: w1157 -> [w1184 w1201]
                    tunnel: w1163 -> [_ w1209]
                    tunnel: w1154 -> [_ w1210]
                    tunnel: [w1181 w1205] -> w1153
                    tunnel: [FALSE w1186] -> w1158
                    tunnel: [0.0 w1197] -> w1155
                    frame False {
                      n731 = Sine(x=w1184) -> (sin(x)=w1182:dbl)
                      n732 = Multiply(x=w1182, y="Osc. amp. (MHz)") -> (x*y=w1181:dbl)
                    }
                    frame True {
                      # "trap position goes from 0 to 1 (0 is when it is furthest away, 1 is when closest)\nso we want to test for tether only when farther away, or x < 1"
                      # "quit if taking too long"
                      # "oscillate the trap"
                      # "Test for tether"
                      n733 = local read "Vec Mean of T1 T2"() -> (w1185:dbl[])
                      "Trigger Signal" <- w1185
                      n734 = Cosine(x=w1201) -> (cos(x)=w1213:dbl)
                      n735 = Subtract(x=w1210, y=w1209) -> (x-y=w1208:dbl)
                      n736 = Decrement(x=w1213) -> (x-1=w1212:dbl)
                      n737 = Subtract(x=w1208, y="Closest Delta (MHz)") -> (x-y=w1206:dbl)
                      n738 = Divide(x=w1212, y=-2.0) -> (x/y=w1196:dbl)
                      n739 = Greater?(x=w1185, y="Stop F (pN)") -> (0:w1203:bool[])
                      n740 = Multiply(x=w1196, y=w1206) -> (x*y=w1205:dbl)
                      n741 = Less?(x=w1196, y="Fish mask thresh") -> (x < y?=w1195:bool)
                      n742 = Boolean To (0,1)(Boolean=w1195) -> (0, 1=w1193:i16)
                      n743 = Multiply(x=w1193, y=w1185) -> (x*y=w1192:dbl[])
                      n744 = Divide(x=w1201, y=6.283185307179586) -> (x/y=w1200:dbl)
                      n745 = Round Toward +Infinity(x=w1200) -> (ceil(x): smallest int >= x=w1197:dbl)
                      "Attempts" <- w1197
                      n746 = Greater?(x=w1192, y="Stop F (pN) (mask)") -> (0:w1190:bool[])
                      n747 = Or Array Elements(Boolean array=w1203) -> (logical OR=w1188:bool)
                      n748 = Or Array Elements(Boolean array=w1190) -> (logical OR=w1187:bool)
                      n749 = Greater?(x=w1197, y="Attempt Limit") -> (0:w1199:bool)
                      n750 = case shown="True" w1199 {
                        frame False {
                        }
                        frame True {
                          n751 = local write "Fish for Tether"(FALSE ("Fish for Tether")) -> ()
                          n752 = call <vilib>:"Beep.vi"() -> ()  [unwired: 3 in, 9 out]
                          n753 = local read "Messages"() -> (w1215:string)
                          n754 = call "Update messages.vi"("Message to add"="Tether fishing timeout." ("Messages"), "Old message string"=w1215) -> ("New message string"=→"Messages":string)
                        }
                      }
                      n755 = Select(t=w1188, s="Normal (on) or masked test (off)", f=w1187) -> (s? t:f=w1186:bool)
                    }
                  }
                  n756 = local read "BD 2 Frequency 1 (MHz)"() -> (w1162:dbl)
                  n757 = Select(t=w1163, s="Scan axis 2", f=w1162) -> (s? t:f=w1166:dbl)
                  n758 = Add(x=w1153, y=w1166) -> (x+y=w1160:dbl)
                  n759 = Select(t=w1160, s="Scan axis 2", f=w1163) -> (s? t:f=w1169:dbl)
                  n760 = Select(t=w1162, s="Scan axis 2", f=w1160) -> (s? t:f=w1168:dbl)
                  n761 = local read "BD 2 Frequency 2 (MHz)"() -> (w1171:dbl)
                  n762 = local read "BD 2 Frequency 3 (MHz)"() -> (w1170:dbl)
                  n763 = local read "Y RF Frequency Limits (MHz)"() -> (w1164:T16)
                  n764 = local read "X RF Frequency Limits (MHz)"() -> (w1165:T16)
                  n765 = local read "BD 1 Frequency 3 (MHz)"() -> (w1172:dbl)
                  n766 = call "set RF board frequency - interlace.vi"("Board 2 Frequency Limits"=w1164, "Board 1 Frequency Limits"=w1165, "FPGA VI Reference In"=w1159, "Board 2 Frequency 3 (MHz)"=w1170, "Board 1 Frequency 3 (MHz)"=w1172, "Board 2 Frequency 2 (MHz)"=w1171, "Board 2 Frequency 1 (MHz)"=w1168, "Board 1 Frequency 2 (MHz)"=w1154, "Board 1 Frequency 1  (MHz)"=w1169) -> ()  [unwired: 1 in, 2 out]
                }
                frame #1 {
                  n767 = And(x=w1223, y=w1220) -> (x .and. y?=w1222:bool)
                  n768 = case "Only if were fishing and now formed tether" shown="True" w1222 {
                    tunnel: w1221 -> [w1225 w1240]
                    tunnel: [w1224 w1239] -> w1219
                    tunnel: w1218 -> [_ w1235]
                    frame False {
                      n769 = local read "Fish for Tether"() -> (w1224:bool)
                      n770 = case shown="False" w1224 {
                        tunnel: w1225 -> [w1226 _]
                        frame False {
                          n771 = property on="BD 1 Frequency 1 (MHz)" class="DigNum (strict)"("Val(Sgnl)"=w1226) -> ()  [unwired: 2 in, 2 out]
                        }
                        frame True {
                        }
                      }
                    }
                    frame True {
                      w1239 = FALSE ("Fish for Tether")
                      n772 = call <vilib>:"Beep.vi"() -> ()  [unwired: 3 in, 9 out]
                      n773 = Number To Decimal String(number=w1235, width (-)=i16 1) -> (decimal integer string=w1233:string)
                      n774 = Concatenate Strings("Formed tether in ", w1233, " attempt(s)." ("string")) -> (w1230:string)
                      n775 = local read "Messages"() -> (w1237:string)
                      n776 = local write "Fish for Tether"(w1239) -> ()
                      n777 = call "Update messages.vi"("Message to add"=w1230, "Old message string"=w1237) -> ("New message string"=w1236:string)
                      n778 = local write "Messages"(w1236) -> ()
                      n779 = Get Date/Time In Seconds() -> (seconds since 1Jan1904=→"Time tether formed":timestamp)
                      n780 = local read "Flow ON during cal?"() -> (w1227:bool)
                      n781 = property on="Sample Channel\nFlow" class="Bool (strict)"("Val(Sgnl)"=w1227) -> (error out=w1228:errorcluster)  [unwired: 2 in, 1 out]
                      n782 = case shown="\"2\", \"3\", \"4\", \"5\", \"6\"" "Then..." {
                        selector: "Then..." -> [_ w1243]